vi "Dresden R2R Sputter 03.02.2018 IY24.vi"() -> ()   [LabVIEW 2009] (continued)
          }
          frame #1 {
            n10291 = local read "Ch2_Mp_do"() -> (w17010:bool)
            n10292 = local read "Ch2_Mp_di"() -> (w17011:bool)
            n10293 = Exclusive Or(1:w17010, 2:w17011) -> (0:w17027:bool)
            n10294 = feedback #399() -> (w17028:bool)  [unwired: 1 in]
            n10295 = case shown="True" w17027 {
              tunnel: [TRUE FALSE] -> w17029
              tunnel: w17028 -> [_ w17070]
              tunnel: [FALSE w17067] -> w17009
              frame #0 {
              }
              frame #1 {
                n10296 = call "Elapsed Time104"("Reset"=w17070) -> ("Elapsed Time (s)"=w17069:dbl)  [unwired: 11 in, 7 out]
                n10297 = Greater?(x=w17069, y=5.0) -> (0:w17067:bool)
              }
            }
            n10298 = local write "Ch2_Mp_fail"(w17009) -> ()
            n10299 = local read "Ch2_Tp_bv_do"() -> (w17007:bool)
            n10300 = local read "Ch2_Tp_bv_di"() -> (w17008:bool)
            n10301 = Exclusive Or(1:w17007, 2:w17008) -> (0:w17026:bool)
            n10302 = feedback #400() -> (w17025:bool)  [unwired: 1 in]
            n10303 = case shown="True" w17026 {
              tunnel: [TRUE FALSE] -> w17024
              tunnel: w17025 -> [_ w17063]
              tunnel: [FALSE w17060] -> w17006
              frame #0 {
              }
              frame #1 {
                n10304 = call "Elapsed Time105"("Reset"=w17063) -> ("Elapsed Time (s)"=w17062:dbl)  [unwired: 11 in, 7 out]
                n10305 = Greater?(x=w17062, y=5.0) -> (0:w17060:bool)
              }
            }
            n10306 = local write "Ch2_Tp_bv_fail"(w17006) -> ()
            n10307 = local read "Ch2_Bg_bv_di"() -> (w17005:bool)
            n10308 = local read "Ch2_Bg_bv_do"() -> (w17004:bool)
            n10309 = Exclusive Or(1:w17004, 2:w17005) -> (0:w17021:bool)
            n10310 = feedback #401() -> (w17022:bool)  [unwired: 1 in]
            n10311 = case shown="True" w17021 {
              tunnel: [TRUE FALSE] -> w17023
              tunnel: w17022 -> [_ w17056]
              tunnel: [FALSE w17053] -> w16995
              frame #0 {
              }
              frame #1 {
                n10312 = call "Elapsed Time106"("Reset"=w17056) -> ("Elapsed Time (s)"=w17055:dbl)  [unwired: 11 in, 7 out]
                n10313 = Greater?(x=w17055, y=5.0) -> (0:w17053:bool)
              }
            }
            n10314 = local write "ch2_bg_bv_fail_top"(w16995) -> ()
            n10315 = local write "Ch2_Bg_bv_fail"(w16995) -> ()
            n10316 = local read "Ch2_Ch_vbv_do"() -> (w17003:bool)
            n10317 = local read "Ch2_Ch_vbv_di"() -> (w16996:bool)
            n10318 = Exclusive Or(1:w17003, 2:w16996) -> (0:w17020:bool)
            n10319 = feedback #402() -> (w17019:bool)  [unwired: 1 in]
            n10320 = case shown="True" w17020 {
              tunnel: [TRUE FALSE] -> w17018
              tunnel: w17019 -> [_ w17049]
              tunnel: [FALSE w17046] -> w17002
              frame #0 {
              }
              frame #1 {
                n10321 = call "Elapsed Time107"("Reset"=w17049) -> ("Elapsed Time (s)"=w17048:dbl)  [unwired: 11 in, 7 out]
                n10322 = Greater?(x=w17048, y=5.0) -> (0:w17046:bool)
              }
            }
            n10323 = local write "Ch2_Ch_vbv_fail"(w17002) -> ()
            n10324 = local read "Ch2_Pl_vbv_do"() -> (w16999:bool)
            n10325 = local read "Ch2_Pl_vbv_di"() -> (w17000:bool)
            n10326 = Exclusive Or(1:w16999, 2:w17000) -> (0:w17017:bool)
            n10327 = feedback #403() -> (w17016:bool)  [unwired: 1 in]
            n10328 = case shown="True" w17017 {
              tunnel: [TRUE FALSE] -> w17015
              tunnel: w17016 -> [_ w17042]
              tunnel: [FALSE w17039] -> w17001
              frame #0 {
              }
              frame #1 {
                n10329 = call "Elapsed Time109"("Reset"=w17042) -> ("Elapsed Time (s)"=w17041:dbl)  [unwired: 11 in, 7 out]
                n10330 = Greater?(x=w17041, y=5.0) -> (0:w17039:bool)
              }
            }
            n10331 = local write "Ch2_Pl_vbv_fail"(w17001) -> ()
            n10332 = local read "Ch2_Cc_on_off_di"() -> (w16998:bool)
            n10333 = local read "Ch2_Cc_on_off_do"() -> (w16997:bool)
            n10334 = feedback #404() -> (w17013:bool)  [unwired: 1 in]
            n10335 = Exclusive Or(1:w16997, 2:w16998) -> (0:w17014:bool)
            n10336 = case shown="True" w17014 {
              tunnel: [TRUE FALSE] -> w17012
              tunnel: w17013 -> [_ w17035]
              tunnel: [FALSE w17032] -> w16994
              frame #0 {
              }
              frame #1 {
                n10337 = call "Elapsed Time111"("Reset"=w17035) -> ("Elapsed Time (s)"=w17034:dbl)  [unwired: 11 in, 7 out]
                n10338 = Greater?(x=w17034, y=5.0) -> (0:w17032:bool)
              }
            }
            n10339 = local write "ch2_cc_fail_top"(w16994) -> ()
            n10340 = local write "Ch2_Ch_cc_fail"(w16994) -> ()
          }
        }
        n10341 = case shown="False" w16923 {
          frame #0 {
            n10342 = local read "Ch2_trns_gv_bp2_do"() -> (w16927:bool)
            n10343 = local read "Ch2_trns_gv_bp2_di"() -> (w16928:bool)
            n10344 = Exclusive Or(1:w16927, 2:w16928) -> (0:w16929:bool)
            n10345 = feedback #405() -> (w16930:bool)  [unwired: 1 in]
            n10346 = case shown="True" w16929 {
              tunnel: [TRUE FALSE] -> w16931
              tunnel: w16930 -> [_ w16937]
              tunnel: [FALSE w16934] -> w16926
              frame #0 {
              }
              frame #1 {
                n10347 = call "Elapsed Time152"("Reset"=w16937) -> ("Elapsed Time (s)"=w16936:dbl)  [unwired: 11 in, 7 out]
                n10348 = Greater?(x=w16936, y=5.0) -> (0:w16934:bool)
              }
            }
            n10349 = local write "Ch2_Trns_gv_bp2_fail"(w16926) -> ()
            n10350 = local write "Ch2_trns_gv_bp2_fail_top"(w16926) -> ()
            n10351 = local write "ch2_trns_gv_bp2_fail_front"(w16926) -> ()
          }
          frame #1 {
            w16939 = TRUE ("Ch2_Trns_gv_bp2_fail")
            n10352 = local write "Ch2_trns_gv_bp2_fail_top"(w16939) -> ()
            n10353 = local write "ch2_trns_gv_bp2_fail_front"(w16939) -> ()
            n10354 = local write "Ch2_Trns_gv_bp2_fail"(w16939) -> ()
          }
        }
        n10355 = case shown="False" w16922 {
          frame #0 {
          }
          frame #1 {
            w16925 = TRUE ("Bp_bv_fail(ch2)L")
            n10356 = local write "Ch2_Trns_gv_bp2_fail"(w16925) -> ()
            n10357 = local write "Ch2_Trns_gv_bp_fail"(w16925) -> ()
            n10358 = local write "Ch2_Bp_bv_fail_R"(w16925) -> ()
            n10359 = local write "Ch2_Bp_bv_fail_L"(w16925) -> ()
          }
        }
      }
    }
    n10360 = Wait Until Next ms Multiple(millisecond multiple=u32 300) -> ()  [unwired: 1 out]
  }
  n10361 = while {
    tunnel: [w17082] -> w782
    tunnel: [w17081] -> w781
    tunnel: w748 -> [w17074]
    tunnel: w747 -> [w17073]
    tunnel: "milliseconds to wait" -> [w17072]
    i -> [w17075]
    stop <- FALSE stop-if-true
    n10362 = stacked-sequence {
      tunnel: [w17087 _] -> w17082
      tunnel: [w17086 _] -> w17081
      tunnel: w17074 -> [w17085 _]
      tunnel: w17073 -> [w17084 _]
      tunnel: w17072 -> [w17083 _]
      frame #0 {
        n10363 = stacked-sequence {
          tunnel: w17085 -> [w17095 _ _ _ _ _]
          tunnel: w17084 -> [w17090 _ _ _ _ _]
          tunnel: [_ _ _ _ w17181 _] -> w17087
          tunnel: [_ _ _ _ w17180 _] -> w17086
          tunnel: w17083 -> [_ w17136 _ w17165 _ w17205]
          frame #0 {
            # "Digital I/O & Analog \nOutput Part"
            n10364 = call-poly <vilib>:"MB Serial Master Query (poly).vi"("VISA resource name"=w17095, "Starting Address"=u16 0, "Quantity"=u16 8, "error in"=w17090, "Serial Parameters"=T39 {"Mode"=enum."RTU", "Slave Address"=1}) -> ("VISA resource name out"=w17094:refnum<visa-resource-name>, "Discrete Inputs"=w17132:bool[], "error out"=w17093:errorcluster)  [unwired: 1 in, 11 out]
            n10365 = Index Array(array=w17132, index=5) -> (element=→"Cnt_Left_slow_di":bool)
            n10366 = Index Array(array=w17132, index=6) -> (element=→"Cnt_Left_limit_di":bool)
            n10367 = Index Array(array=w17132, index=7) -> (element=→"Cnt_wfs_di":bool)
            n10368 = Index Array(array=w17132, index=0) -> (element=→"Casette_servo_start/stop_di":bool)
            n10369 = Index Array(array=w17132, index=1) -> (element=→"Casette_servo_left_direction_di":bool)
            n10370 = Index Array(array=w17132, index=2) -> (element=→"Tension_controllers_start/stop_di":bool)
            n10371 = Index Array(array=w17132, index=3) -> (element=→"Cnt_Right_limit_di":bool)
            n10372 = Index Array(array=w17132, index=4) -> (element=→"Cnt_Right_slow_di":bool)
            n10373 = local read "Load_dido"() -> (w17089:bool)
            n10374 = case shown="True" w17089 {
              frame #0 {
              }
              frame #1 {
                n10375 = Wait (ms)(milliseconds to wait=u32 2000) -> ()  [unwired: 1 out]
              }
            }
            n10376 = call-poly <vilib>:"MB Serial Master Query (poly).vi"("VISA resource name"=w17094, "Starting Address"=u16 0, "Quantity"=u16 8, "error in"=w17093, "Serial Parameters"=T39 {"Mode"=enum."RTU", "Slave Address"=2}) -> ("VISA resource name out"=w17092:refnum<visa-resource-name>, "Discrete Inputs"=w17113:bool[], "error out"=w17091:errorcluster)  [unwired: 1 in, 11 out]
            n10377 = Index Array(array=w17113, index=5) -> (element=→"Cnt_MW2_Temperature_di":bool)
            n10378 = Index Array(array=w17113, index=6) -> (element=→"Cnt_Di_2_6":bool)
            n10379 = Index Array(array=w17113, index=7) -> (element=→"Cnt_Di_2_7":bool)
            n10380 = Index Array(array=w17113, index=0) -> (element=→"Cnt_Dcps_sw1_di":bool)
            n10381 = Index Array(array=w17113, index=1) -> (element=→"Cnt_Dcps_sw2_di":bool)
            n10382 = Index Array(array=w17113, index=2) -> (element=→"Cnt_Dcps_sw3_di":bool)
            n10383 = Index Array(array=w17113, index=3) -> (element=→"Cnt_Dcps_sw4_di":bool)
            n10384 = Index Array(array=w17113, index=4) -> (element=→"Cnt_MW1_Temperature_di":bool)
          }
          frame #1 {
            n10385 = Wait (ms)(milliseconds to wait=w17136) -> ()  [unwired: 1 out]
          }
          frame #2 {
            n10386 = Build Array("Cnt_Dcps_sw1_do", "Cnt_Dcps_sw2_do", "Cnt_Dcps_sw3_do", "Cnt_Dcps_sw4_do", "Cnt_Do_2_4", "Cnt_Do_2_5", "Cnt_Do_2_6", "Cnt_Do_2_7") -> (w17155:bool[])
            n10387 = call-poly <vilib>:"MB Serial Master Query (poly).vi"("VISA resource name"=w17145, "Starting Address"=u16 320, "Coils"=w17155, "error in"=w17144, "Serial Parameters"=T39 {"Mode"=enum."RTU", "Slave Address"=2}) -> ("VISA resource name out"=w17143:refnum<visa-resource-name>, "error out"=w17142:errorcluster)  [unwired: 1 in, 12 out]
            n10388 = Build Array("Casette_servo_start/stop_do", "Casette_servo_left_direction_do", "Tension_controllers_start/stop_do", "Cnt_Right_limit_do", "Cnt_Right_slow_do", "Cnt_Left_slow_do", "Cnt_Left_limit_do", "Cnt_Do_Buzzer") -> (w17146:bool[])
            n10389 = call-poly <vilib>:"MB Serial Master Query (poly).vi"("VISA resource name"=w17143, "Starting Address"=u16 320, "Coils"=w17146, "error in"=w17142, "Serial Parameters"=T39 {"Mode"=enum."RTU", "Slave Address"=1}) -> ("VISA resource name out"=w17141:refnum<visa-resource-name>, "error out"=w17140:errorcluster)  [unwired: 1 in, 12 out]
          }
          frame #3 {
            n10390 = Wait (ms)(milliseconds to wait=w17165) -> ()  [unwired: 1 out]
          }
          frame #4 {
            n10391 = Or(x="Cassette_servo_speed_set", y="Cassette_servo_speed_auto_set") -> (x .or. y?=w17166:bool)
            n10392 = Build Array(FALSE, "Cntr_AO1 _set", w17166, "Tension_controller1_set", "Tension_controller2_set") -> (w17177:bool[])
            n10393 = Boolean Array To Number(Boolean array=w17177) -> (number=w17179:u32)
            n10394 = Mantissa & Exponent(0:w17179) -> (2:w17176:dbl)  [unwired: 1 out]
            n10395 = case shown="3" w17176 {
              tunnel: [u16 0 ("Starting Address") u16 1184 ("Starting Address") u16 1185 ("Starting Address") u16 1186 ("Starting Address") u16 1187 ("Starting Address")] -> w17182
              tunnel: [u16 0 ("Ao_1_3") "AO1" "Cassette_servo_speed_value" w17193 w17200] -> w17175
              frame #0 {
              }
              frame #1 {
              }
              frame #2 {
                n10396 = local write "Cassette_servo_speed_auto_set"(FALSE ("Cassette_servo_speed_auto_set")) -> ()
              }
              frame #3 {
                n10397 = local write "Tension_controller1_set"(FALSE ("Tension_controller1_set")) -> ()
                n10398 = Divide(x=4096.0, y=10.0) -> (x/y=w17192:dbl)
                n10399 = Multiply(x=w17192, y="Tension_controller1_set_value") -> (x*y=w17193:dbl)
              }
              frame #4 {
                n10400 = Divide(x=4096.0, y=10.0) -> (x/y=w17201:dbl)
                n10401 = Multiply(x=w17201, y="Tension_controller2_set_value") -> (x*y=w17200:dbl)
                n10402 = local write "Tension_controller2_set"(FALSE ("Tension_controller2_set")) -> ()
              }
            }
            n10403 = Build Array(w17175) -> (w17174:dbl[])
            n10404 = call-poly <vilib>:"MB Serial Master Query (poly).vi"("VISA resource name"=w17170, "Starting Address"=w17182, "Registers"=w17174, "error in"=w17169, "Serial Parameters"=T39 {"Mode"=enum."RTU", "Slave Address"=4}) -> ("VISA resource name out"=w17181:refnum<visa-resource-name>, "error out"=w17180:errorcluster)  [unwired: 1 in, 12 out]
          }
          frame #5 {
            n10405 = Wait (ms)(milliseconds to wait=w17205) -> ()  [unwired: 1 out]
          }
        }
      }
      frame #1 {
        n10406 = local read "Fail_moxa_cntr_digital1"() -> (w17207:bool)
        n10407 = local read "Fail_moxa_cntr_digital2"() -> (w17206:bool)
        n10408 = case shown="False" w17207 {
          frame #0 {
          }
          frame #1 {
          }
        }
        n10409 = case shown="False" w17206 {
          frame #0 {
          }
          frame #1 {
          }
        }
      }
    }
    n10410 = Wait Until Next ms Multiple(millisecond multiple=u32 100) -> ()  [unwired: 1 out]
    n10411 = In Range and Coerce(upper limit=4, x=w17075, lower limit=0) -> (In Range?=w17077:bool)  [unwired: 1 out]
    "Load_dido" <- w17077
    n10412 = case shown="True" w17077 {
      frame #0 {
      }
      frame #1 {
        "Semi" <- FALSE ("Semi")
      }
    }
  }
  n10413 = while {
    stop <- FALSE stop-if-true
    n10414 = Wait Until Next ms Multiple(millisecond multiple=u32 100) -> ()  [unwired: 1 out]
    n10415 = case shown="True" "Start_roll" {
      tunnel: "Timer Reset Roll 2" -> [_ w17213]
      frame #0 {
      }
      frame #1 {
        n10416 = Increment(x="Target Chamber Sensor") -> (x+1=w17214:u16)
        n10417 = case shown="4" w17214 {
          tunnel: w17213 -> [_ w17216 w17313 w17410 w17507]
          frame #0 {
          }
          frame #1 {
            n10418 = case shown="\"Right to Left\"" "Roll_side_select" {
              tunnel: w17216 -> [_ w17265]
              tunnel: w17216 -> [w17218 _]
              frame #0 {
                n10419 = stacked-sequence {
                  tunnel: w17218 -> [_ _ _ _ w17229 _]
                  frame #0 {
                    n10420 = local read "Output voltage value"() -> (w17221:dbl)
                    n10421 = local write "Ch1_SRV_counterclockwise_direction_do"(TRUE ("Ch2_SRV1_direction_do")) -> ()
                    n10422 = Wait (ms)(milliseconds to wait=u32 10) -> ()  [unwired: 1 out]
                    n10423 = local write "Tension_controller2_set_value"(w17221) -> ()
                    "Actual Lap" <- 0.0 ("Actual Lap")
                    "Actual Length" <- 0.0 ("Actual Region")
                  }
                  frame #1 {
                    n10424 = local write "Tension_controller2_set"(TRUE ("Tension_controller2_set")) -> ()
                  }
                  frame #2 {
                    n10425 = Wait (ms)(milliseconds to wait=u32 10) -> ()  [unwired: 1 out]
                  }
                  frame #3 {
                    n10426 = local write "Tension_controllers_start/stop_do"(TRUE ("Tension_controllers_start/stop_do")) -> ()
                    n10427 = local write "Ch1_SRV_start_stop_do"(TRUE ("Ch2_SRV1_start_stop_do")) -> ()
                    n10428 = Wait (ms)(milliseconds to wait=u32 10) -> ()  [unwired: 1 out]
                  }
                  frame #4 {
                    n10429 = while {
                      tunnel: w17229 -> [w17231]
                      stop <- w17233 stop-if-true
                      n10430 = call "Elapsed Time140"("Reset"=w17231) -> ("Elapsed Time (s)"=w17235:dbl)  [unwired: 11 in, 7 out]
                      "Elapsed Time (s) 2" <- w17235
                      n10431 = Wait Until Next ms Multiple(millisecond multiple=u32 10) -> ()  [unwired: 1 out]
                      n10432 = local read "Start_roll"() -> (w17238:bool)
                      n10433 = Greater Or Equal?(x=w17235, y="Left to Right") -> (x >= y?=w17232:bool)
                      n10434 = case shown="False" FALSE {
                        frame #0 {
                          n10435 = local read "To Right Volt"() -> (w17240:dbl)
                          n10436 = local write "Tension_controller2_set_value"(w17240) -> ()
                          n10437 = local write "Tension_controller2_set"(TRUE ("Tension_controller2_set")) -> ()
                        }
                        frame #1 {
                          n10438 = stacked-sequence {
                            frame #0 {
                              n10439 = local read "Actual Diameter"() -> (w17245:dbl)
                              n10440 = local read "Web Thickness"() -> (w17254:dbl)
                              n10441 = local read "Actual Diameter"() -> (w17248:dbl)
                              n10442 = local read "Actual Lap"() -> (w17246:dbl)
                              n10443 = Multiply(x=w17254, y=0.002) -> (x*y=w17255:dbl)
                              n10444 = Increment(x=w17246) -> (x+1=w17244:dbl)
                              n10445 = Add(x=w17245, y=w17255) -> (x+y=w17253:dbl)
                              n10446 = local read "Actual Length"() -> (w17247:dbl)
                              n10447 = Multiply(x=w17248, y=3.14) -> (x*y=w17250:dbl)
                              n10448 = local write "Actual Diameter"(w17253) -> ()
                              n10449 = local write "Actual Lap"(w17244) -> ()
                              n10450 = Divide(x=w17250, y=1000.0) -> (x/y=w17252:dbl)
                              n10451 = Add(x=w17252, y=w17247) -> (x+y=w17243:dbl)
                              n10452 = disable-structure shown="Disabled" {
                                frame #0 {
                                n10453 = local read "Output voltage value"() -> (w17259:dbl)
                                n10454 = local read "Set voltage value"() -> (w17258:dbl)
                                n10455 = Subtract(x=w17259, y=w17258) -> (x-y=w17257:dbl)
                                n10456 = local write "Output voltage value"(w17257) -> ()
                                }
                                frame #1 {
                                }
                              }
                              n10457 = Wait (ms)(milliseconds to wait=u32 10) -> ()  [unwired: 1 out]
                              n10458 = local write "Actual Length"(w17243) -> ()
                            }
                            frame #1 {
                              n10459 = local read "Output voltage value"() -> (w17260:dbl)
                              n10460 = Wait (ms)(milliseconds to wait=u32 10) -> ()  [unwired: 1 out]
                              n10461 = local write "Tension_controller2_set_value"(w17260) -> ()
                            }
                            frame #2 {
                              n10462 = local write "Tension_controller2_set"(TRUE ("Tension_controller2_set")) -> ()
                            }
                          }
                        }
                      }
                      n10463 = Not(x=w17238) -> (.not. x?=w17236:bool)
                      n10464 = case shown="True" w17232 {
                        frame #0 {
                        }
                        frame #1 {
                          n10465 = local write "Ch1_SRV_start_stop_do"(FALSE ("Ch2_SRV1_start_stop_do")) -> ()
                        }
                      }
                      n10466 = Or(x=w17232, y=w17236) -> (x .or. y?=w17233:bool)
                    }
                  }
                  frame #5 {
                    n10467 = local write "Test_stop"(TRUE ("Test_stop")) -> ()
                    n10468 = Wait (ms)(milliseconds to wait=u32 10) -> ()  [unwired: 1 out]
                  }
                }
              }
              frame #1 {
                n10469 = stacked-sequence {
                  tunnel: w17265 -> [_ _ _ _ w17276 _]
                  frame #0 {
                    n10470 = local read "Output voltage value"() -> (w17266:dbl)
                    n10471 = local write "Ch1_SRV_counterclockwise_direction_do"(FALSE ("Ch2_SRV1_direction_do")) -> ()
                    n10472 = local write "Actual Lap"(0.0 ("Actual Lap")) -> ()
                    n10473 = local write "Actual Length"(0.0 ("Actual Region")) -> ()
                    n10474 = Wait (ms)(milliseconds to wait=u32 10) -> ()  [unwired: 1 out]
                    n10475 = local write "Tension_controller1_set_value"(w17266) -> ()
                  }
                  frame #1 {
                    n10476 = local write "Tension_controller1_set"(TRUE ("Tension_controller2_set")) -> ()
                  }
                  frame #2 {
                    n10477 = Wait (ms)(milliseconds to wait=u32 10) -> ()  [unwired: 1 out]
                  }
                  frame #3 {
                    n10478 = local write "Tension_controllers_start/stop_do"(TRUE ("Tension_controllers_start/stop_do")) -> ()
                    n10479 = local write "Ch1_SRV_start_stop_do"(TRUE ("Ch2_SRV1_start_stop_do")) -> ()
                    n10480 = Wait (ms)(milliseconds to wait=u32 10) -> ()  [unwired: 1 out]
                  }
                  frame #4 {
                    n10481 = while {
                      tunnel: w17276 -> [w17278]
                      stop <- w17280 stop-if-true
                      n10482 = Wait Until Next ms Multiple(millisecond multiple=u32 10) -> ()  [unwired: 1 out]
                      n10483 = call "Elapsed Time138"("Reset"=w17278) -> ("Elapsed Time (s)"=w17282:dbl)  [unwired: 11 in, 7 out]
                      "Elapsed Time (s)" <- w17282
                      n10484 = case shown="False" FALSE {
                        frame #0 {
                          n10485 = local read "To Left Volt"() -> (w17287:dbl)
                          n10486 = local write "Tension_controller1_set"(TRUE ("Tension_controller2_set")) -> ()
                          n10487 = local write "Tension_controller1_set_value"(w17287) -> ()
                        }
                        frame #1 {
                          n10488 = stacked-sequence {
                            frame #0 {
                              n10489 = local read "Actual Diameter"() -> (w17295:dbl)
                              n10490 = local read "Actual Diameter"() -> (w17292:dbl)
                              n10491 = local read "Web Thickness"() -> (w17301:dbl)
                              n10492 = local read "Actual Lap"() -> (w17293:dbl)
                              n10493 = Increment(x=w17293) -> (x+1=w17291:dbl)
                              n10494 = local read "Actual Length"() -> (w17294:dbl)
                              n10495 = Multiply(x=w17301, y=0.002) -> (x*y=w17302:dbl)
                              n10496 = Multiply(x=w17295, y=3.14) -> (x*y=w17297:dbl)
                              n10497 = Add(x=w17292, y=w17302) -> (x+y=w17300:dbl)
                              n10498 = local write "Actual Lap"(w17291) -> ()
                              n10499 = Divide(x=w17297, y=1000.0) -> (x/y=w17299:dbl)
                              n10500 = local write "Actual Diameter"(w17300) -> ()
                              n10501 = Add(x=w17299, y=w17294) -> (x+y=w17290:dbl)
                              n10502 = disable-structure shown="Disabled" {
                                frame #0 {
                                n10503 = local read "Output voltage value"() -> (w17306:dbl)
                                n10504 = local read "Set voltage value"() -> (w17305:dbl)
                                n10505 = Subtract(x=w17306, y=w17305) -> (x-y=w17304:dbl)
                                n10506 = local write "Output voltage value"(w17304) -> ()
                                }
                                frame #1 {
                                }
                              }
                              n10507 = local write "Actual Length"(w17290) -> ()
                              n10508 = Wait (ms)(milliseconds to wait=u32 10) -> ()  [unwired: 1 out]
                            }
                            frame #1 {
                              n10509 = local read "Output voltage value"() -> (w17307:dbl)
                              n10510 = local write "Tension_controller1_set_value"(w17307) -> ()
                              n10511 = Wait (ms)(milliseconds to wait=u32 10) -> ()  [unwired: 1 out]
                            }
                            frame #2 {
                              n10512 = local write "Tension_controller1_set"(TRUE ("Tension_controller2_set")) -> ()
                              "Actual Region led" <- TRUE ("Actual Region")
                            }
                          }
                        }
                      }
                      n10513 = Greater Or Equal?(x=w17282, y="Right to Left") -> (x >= y?=w17279:bool)
                      n10514 = local read "Start_roll"() -> (w17285:bool)
                      n10515 = Not(x=w17285) -> (.not. x?=w17283:bool)
                      n10516 = Or(x=w17279, y=w17283) -> (x .or. y?=w17280:bool)
                      n10517 = case shown="True" w17279 {
                        frame #0 {
                        }
                        frame #1 {
                          n10518 = local write "Ch1_SRV_start_stop_do"(FALSE ("Ch2_SRV1_start_stop_do")) -> ()
                        }
                      }
                    }
                  }
                  frame #5 {
                    n10519 = local write "Test_stop"(TRUE ("Test_stop")) -> ()
                    n10520 = Wait (ms)(milliseconds to wait=u32 10) -> ()  [unwired: 1 out]
                  }
                }
              }
            }
          }
          frame #2 {
            n10521 = local read "Roll_side_select"() -> (w17314:enum32{"Left to Right", "Right to Left"})
            n10522 = case shown="\"Right to Left\"" w17314 {
              tunnel: w17313 -> [_ w17362]
              tunnel: w17313 -> [w17315 _]
              frame #0 {
                n10523 = stacked-sequence {
                  tunnel: w17315 -> [_ _ _ _ w17326 _]
                  frame #0 {
                    n10524 = local read "Output voltage value"() -> (w17318:dbl)
                    n10525 = local write "Ch2_SRV_counterclockwise_direction_do"(TRUE ("Ch2_SRV1_direction_do")) -> ()
                    n10526 = local write "Actual Lap"(0.0 ("Actual Lap")) -> ()
                    n10527 = local write "Actual Length"(0.0 ("Actual Region")) -> ()
                    n10528 = Wait (ms)(milliseconds to wait=u32 10) -> ()  [unwired: 1 out]
                    n10529 = local write "Tension_controller2_set_value"(w17318) -> ()
                  }
                  frame #1 {
                    n10530 = local write "Tension_controller2_set"(TRUE ("Tension_controller2_set")) -> ()
                  }
                  frame #2 {
                    n10531 = Wait (ms)(milliseconds to wait=u32 10) -> ()  [unwired: 1 out]
                  }
                  frame #3 {
                    n10532 = local write "Tension_controllers_start/stop_do"(TRUE ("Tension_controllers_start/stop_do")) -> ()
                    n10533 = local write "Ch2_SRV_start_stop_do"(TRUE ("Ch2_SRV1_start_stop_do")) -> ()
                    n10534 = Wait (ms)(milliseconds to wait=u32 10) -> ()  [unwired: 1 out]
                  }
                  frame #4 {
                    n10535 = while {
                      tunnel: w17326 -> [w17328]
                      stop <- w17330 stop-if-true
                      n10536 = call "Elapsed Time149"("Reset"=w17328) -> ("Elapsed Time (s)"=w17332:dbl)  [unwired: 11 in, 7 out]
                      "Elapsed Time (s) 5" <- w17332
                      n10537 = Wait Until Next ms Multiple(millisecond multiple=u32 10) -> ()  [unwired: 1 out]
                      n10538 = local read "Start_roll"() -> (w17335:bool)
                      n10539 = Greater Or Equal?(x=w17332, y="Left to Right 3") -> (x >= y?=w17329:bool)
                      n10540 = case shown="True" FALSE {
                        frame #0 {
                          n10541 = local read "To Right Volt"() -> (w17337:dbl)
                          n10542 = local write "Tension_controller2_set_value"(w17337) -> ()
                          n10543 = local write "Tension_controller2_set"(TRUE ("Tension_controller2_set")) -> ()
                        }
                        frame #1 {
                          n10544 = stacked-sequence {
                            frame #0 {
                              n10545 = local read "Actual Diameter"() -> (w17344:dbl)
                              n10546 = local read "Web Thickness"() -> (w17351:dbl)
                              n10547 = local read "Actual Diameter"() -> (w17345:dbl)
                              n10548 = local read "Actual Lap"() -> (w17339:dbl)
                              n10549 = Multiply(x=w17351, y=0.002) -> (x*y=w17352:dbl)
                              n10550 = Increment(x=w17339) -> (x+1=w17340:dbl)
                              n10551 = Add(x=w17344, y=w17352) -> (x+y=w17350:dbl)
                              n10552 = local read "Actual Length"() -> (w17341:dbl)
                              n10553 = Multiply(x=w17345, y=3.14) -> (x*y=w17347:dbl)
                              n10554 = local write "Actual Diameter"(w17350) -> ()
                              n10555 = local write "Actual Lap"(w17340) -> ()
                              n10556 = Divide(x=w17347, y=1000.0) -> (x/y=w17349:dbl)
                              n10557 = Add(x=w17349, y=w17341) -> (x+y=w17342:dbl)
                              n10558 = disable-structure shown="Disabled" {
                                frame #0 {
                                n10559 = local read "Output voltage value"() -> (w17356:dbl)
                                n10560 = local read "Set voltage value"() -> (w17355:dbl)
                                n10561 = Subtract(x=w17356, y=w17355) -> (x-y=w17354:dbl)
                                n10562 = local write "Output voltage value"(w17354) -> ()
                                }
                                frame #1 {
                                }
                              }
                              n10563 = Wait (ms)(milliseconds to wait=u32 10) -> ()  [unwired: 1 out]
                              n10564 = local write "Actual Length"(w17342) -> ()
                            }
                            frame #1 {
                              n10565 = local read "Output voltage value"() -> (w17357:dbl)
                              n10566 = Wait (ms)(milliseconds to wait=u32 10) -> ()  [unwired: 1 out]
                              n10567 = local write "Tension_controller2_set_value"(w17357) -> ()
                            }
                            frame #2 {
                              n10568 = local write "Tension_controller2_set"(TRUE ("Tension_controller2_set")) -> ()
                            }
                          }
                        }
                      }
                      n10569 = Not(x=w17335) -> (.not. x?=w17333:bool)
                      n10570 = case shown="True" w17329 {
                        frame #0 {
                        }
                        frame #1 {
                          n10571 = local write "Ch2_SRV_start_stop_do"(FALSE ("Ch2_SRV1_start_stop_do")) -> ()
                        }
                      }
                      n10572 = Or(x=w17329, y=w17333) -> (x .or. y?=w17330:bool)
                    }
                  }
                  frame #5 {
                    n10573 = local write "Test_stop"(TRUE ("Test_stop")) -> ()
                    n10574 = Wait (ms)(milliseconds to wait=u32 10) -> ()  [unwired: 1 out]
                  }
                }
              }
              frame #1 {
                n10575 = stacked-sequence {
                  tunnel: w17362 -> [_ _ _ _ w17373 _]
                  frame #0 {
                    n10576 = local read "Output voltage value"() -> (w17363:dbl)
                    n10577 = local write "Ch2_SRV_counterclockwise_direction_do"(FALSE ("Ch2_SRV1_direction_do")) -> ()
                    n10578 = local write "Actual Lap"(0.0 ("Actual Lap")) -> ()
                    n10579 = local write "Actual Length"(0.0 ("Actual Region")) -> ()
                    n10580 = Wait (ms)(milliseconds to wait=u32 10) -> ()  [unwired: 1 out]
                    n10581 = local write "Tension_controller1_set_value"(w17363) -> ()
                  }
                  frame #1 {
                    n10582 = local write "Tension_controller1_set"(TRUE ("Tension_controller2_set")) -> ()
                  }
                  frame #2 {
                    n10583 = Wait (ms)(milliseconds to wait=u32 10) -> ()  [unwired: 1 out]
                  }
                  frame #3 {
                    n10584 = local write "Tension_controllers_start/stop_do"(TRUE ("Tension_controllers_start/stop_do")) -> ()
                    n10585 = local write "Ch2_SRV_start_stop_do"(TRUE ("Ch2_SRV1_start_stop_do")) -> ()
                    n10586 = Wait (ms)(milliseconds to wait=u32 10) -> ()  [unwired: 1 out]
                  }
                  frame #4 {
                    n10587 = while {
                      tunnel: w17373 -> [w17375]
                      stop <- w17377 stop-if-true
                      n10588 = Wait Until Next ms Multiple(millisecond multiple=u32 10) -> ()  [unwired: 1 out]
                      n10589 = call "Elapsed Time150"("Reset"=w17375) -> ("Elapsed Time (s)"=w17379:dbl)  [unwired: 11 in, 7 out]
                      "Elapsed Time (s) 6" <- w17379
                      n10590 = case shown="True" FALSE {
                        frame #0 {
                          n10591 = local read "To Left Volt"() -> (w17384:dbl)
                          n10592 = local write "Tension_controller1_set"(TRUE ("Tension_controller2_set")) -> ()
                          n10593 = local write "Tension_controller1_set_value"(w17384) -> ()
                        }
                        frame #1 {
                          n10594 = stacked-sequence {
                            frame #0 {
                              n10595 = local read "Actual Diameter"() -> (w17392:dbl)
                              n10596 = local read "Actual Diameter"() -> (w17389:dbl)
                              n10597 = local read "Web Thickness"() -> (w17398:dbl)
                              n10598 = local read "Actual Lap"() -> (w17390:dbl)
                              n10599 = Increment(x=w17390) -> (x+1=w17388:dbl)
                              n10600 = local read "Actual Length"() -> (w17391:dbl)
                              n10601 = Multiply(x=w17398, y=0.002) -> (x*y=w17399:dbl)
                              n10602 = Multiply(x=w17392, y=3.14) -> (x*y=w17394:dbl)
                              n10603 = local write "Actual Lap"(w17388) -> ()
                              n10604 = Add(x=w17389, y=w17399) -> (x+y=w17397:dbl)
                              n10605 = Divide(x=w17394, y=1000.0) -> (x/y=w17396:dbl)
                              n10606 = local write "Actual Diameter"(w17397) -> ()
                              n10607 = Add(x=w17396, y=w17391) -> (x+y=w17387:dbl)
                              n10608 = disable-structure shown="Disabled" {
                                frame #0 {
                                n10609 = local read "Output voltage value"() -> (w17403:dbl)
                                n10610 = local read "Set voltage value"() -> (w17402:dbl)
                                n10611 = Subtract(x=w17403, y=w17402) -> (x-y=w17401:dbl)
                                n10612 = local write "Output voltage value"(w17401) -> ()
                                }
                                frame #1 {
                                }
                              }
                              n10613 = local write "Actual Length"(w17387) -> ()
                              n10614 = Wait (ms)(milliseconds to wait=u32 10) -> ()  [unwired: 1 out]
                            }
                            frame #1 {
                              n10615 = local read "Output voltage value"() -> (w17404:dbl)
                              n10616 = local write "Tension_controller1_set_value"(w17404) -> ()
                              n10617 = Wait (ms)(milliseconds to wait=u32 10) -> ()  [unwired: 1 out]
                            }
                            frame #2 {
                              n10618 = local write "Tension_controller1_set"(TRUE ("Tension_controller2_set")) -> ()
                              "Actual Region led 3" <- TRUE ("Actual Region")
                            }
                          }
                        }
                      }
                      n10619 = Greater Or Equal?(x=w17379, y="Right to Left 3") -> (x >= y?=w17376:bool)
                      n10620 = local read "Start_roll"() -> (w17382:bool)
                      n10621 = Not(x=w17382) -> (.not. x?=w17380:bool)
                      n10622 = Or(x=w17376, y=w17380) -> (x .or. y?=w17377:bool)
                      n10623 = case shown="True" w17376 {
                        frame #0 {
                        }
                        frame #1 {
                          n10624 = local write "Ch2_SRV_start_stop_do"(FALSE ("Ch2_SRV1_start_stop_do")) -> ()
                        }
                      }
                    }
                  }
                  frame #5 {
                    n10625 = local write "Test_stop"(TRUE ("Test_stop")) -> ()
                    n10626 = Wait (ms)(milliseconds to wait=u32 10) -> ()  [unwired: 1 out]
                  }
                }
              }
            }
          }
          frame #3 {
            n10627 = local read "Roll_side_select"() -> (w17411:enum32{"Left to Right", "Right to Left"})
            n10628 = case shown="\"Left to Right\", Default" w17411 {
              tunnel: w17410 -> [_ w17459]
              tunnel: w17410 -> [w17412 _]
              frame #0 {
                n10629 = stacked-sequence {
                  tunnel: w17412 -> [_ _ _ _ w17423 _]
                  frame #0 {
                    n10630 = local read "Output voltage value"() -> (w17415:dbl)
                    n10631 = local write "Ch3_SRV_counterclockwise_direction_do"(TRUE ("Ch2_SRV1_direction_do")) -> ()
                    n10632 = local write "Actual Lap"(0.0 ("Actual Lap")) -> ()
                    n10633 = local write "Actual Length"(0.0 ("Actual Region")) -> ()
                    n10634 = Wait (ms)(milliseconds to wait=u32 10) -> ()  [unwired: 1 out]
                    n10635 = local write "Tension_controller2_set_value"(w17415) -> ()
                  }
                  frame #1 {
                    n10636 = local write "Tension_controller2_set"(TRUE ("Tension_controller2_set")) -> ()
                  }
                  frame #2 {
                    n10637 = Wait (ms)(milliseconds to wait=u32 10) -> ()  [unwired: 1 out]
                  }
                  frame #3 {
                    n10638 = local write "Tension_controllers_start/stop_do"(TRUE ("Tension_controllers_start/stop_do")) -> ()
                    n10639 = local write "Ch3_SRV_start_stop_do"(TRUE ("Ch2_SRV1_start_stop_do")) -> ()
                    n10640 = Wait (ms)(milliseconds to wait=u32 10) -> ()  [unwired: 1 out]
                  }
                  frame #4 {
                    n10641 = while {
                      tunnel: w17423 -> [w17425]
                      stop <- w17427 stop-if-true
                      n10642 = call "Elapsed Time151"("Reset"=w17425) -> ("Elapsed Time (s)"=w17429:dbl)  [unwired: 11 in, 7 out]
                      "Elapsed Time (s) 9" <- w17429
                      n10643 = Wait Until Next ms Multiple(millisecond multiple=u32 10) -> ()  [unwired: 1 out]
                      n10644 = local read "Start_roll"() -> (w17432:bool)
                      n10645 = Greater Or Equal?(x=w17429, y="Left to Right 5") -> (x >= y?=w17426:bool)
                      n10646 = case shown="True" FALSE {
                        frame #0 {
                          n10647 = local read "To Right Volt"() -> (w17434:dbl)
                          n10648 = local write "Tension_controller2_set_value"(w17434) -> ()
                          n10649 = local write "Tension_controller2_set"(TRUE ("Tension_controller2_set")) -> ()
                        }
                        frame #1 {
                          n10650 = stacked-sequence {
                            frame #0 {
                              n10651 = local read "Actual Diameter"() -> (w17441:dbl)
                              n10652 = local read "Web Thickness"() -> (w17448:dbl)
                              n10653 = local read "Actual Diameter"() -> (w17442:dbl)
                              n10654 = local read "Actual Lap"() -> (w17436:dbl)
                              n10655 = Multiply(x=w17448, y=0.002) -> (x*y=w17449:dbl)
                              n10656 = Increment(x=w17436) -> (x+1=w17437:dbl)
                              n10657 = Add(x=w17441, y=w17449) -> (x+y=w17447:dbl)
                              n10658 = local read "Actual Length"() -> (w17438:dbl)
                              n10659 = Multiply(x=w17442, y=3.14) -> (x*y=w17444:dbl)
                              n10660 = local write "Actual Diameter"(w17447) -> ()
                              n10661 = local write "Actual Lap"(w17437) -> ()
                              n10662 = Divide(x=w17444, y=1000.0) -> (x/y=w17446:dbl)
                              n10663 = Add(x=w17446, y=w17438) -> (x+y=w17439:dbl)
                              n10664 = disable-structure shown="Disabled" {
                                frame #0 {
                                n10665 = local read "Output voltage value"() -> (w17453:dbl)
                                n10666 = local read "Set voltage value"() -> (w17452:dbl)
                                n10667 = Subtract(x=w17453, y=w17452) -> (x-y=w17451:dbl)
                                n10668 = local write "Output voltage value"(w17451) -> ()
                                }
                                frame #1 {
                                }
                              }
                              n10669 = Wait (ms)(milliseconds to wait=u32 10) -> ()  [unwired: 1 out]
                              n10670 = local write "Actual Length"(w17439) -> ()
                            }
                            frame #1 {
                              n10671 = local read "Output voltage value"() -> (w17454:dbl)
                              n10672 = Wait (ms)(milliseconds to wait=u32 10) -> ()  [unwired: 1 out]
                              n10673 = local write "Tension_controller2_set_value"(w17454) -> ()
                            }
                            frame #2 {
                              n10674 = local write "Tension_controller2_set"(TRUE ("Tension_controller2_set")) -> ()
                            }
                          }
                        }
                      }
                      n10675 = Not(x=w17432) -> (.not. x?=w17430:bool)
                      n10676 = case shown="True" w17426 {
                        frame #0 {
                        }
                        frame #1 {
                          n10677 = local write "Ch3_SRV_start_stop_do"(FALSE ("Ch2_SRV1_start_stop_do")) -> ()